vi "HFRR ADV v043.vi"() -> ()   [LabVIEW 2025] (continued)
              n2247 = Fract/Exp String To Number(string=w2642) -> (number=w2638:dbl)  [unwired: 3 in, 1 out]
              n2248 = Fract/Exp String To Number(string=w2632) -> (number=w2635:dbl)  [unwired: 3 in, 1 out]
              n2249 = Add(x=w2635, y=0.0) -> (x+y=w2631:dbl)
            }
            n2250 = Delete From Array(array=w2497, index=0) -> (array with subset deleted=w2470:dbl[])  [unwired: 1 in, 1 out]
            n2251 = Delete From Array(array=w2560, index=0) -> (array with subset deleted=w2533:dbl[])  [unwired: 1 in, 1 out]
            n2252 = Delete From Array(array=w2540, index=0) -> (array with subset deleted=w2528:dbl[])  [unwired: 1 in, 1 out]
            n2253 = Delete From Array(array=w2558, index=0) -> (array with subset deleted=w2559:dbl[])  [unwired: 1 in, 1 out]
            n2254 = call-poly <vilib>:"Mean.vi"("X"=w2470) -> ("mean"=→"КОФ2 4":dbl)  [unwired: 1 out]
            n2255 = call-poly <vilib>:"Mean.vi"("X"=w2533) -> ("mean"=→"КОФ3":dbl)  [unwired: 1 out]
            n2256 = call-poly <vilib>:"Mean.vi"("X"=w2528) -> ("mean"=→"CP3":dbl)  [unwired: 1 out]
            n2257 = Delete From Array(array=w2522, index=0) -> (array with subset deleted=w2449:dbl[])  [unwired: 1 in, 1 out]
            n2258 = Delete From Array(array=w2461, index=0) -> (array with subset deleted=w2448:dbl[])  [unwired: 1 in, 1 out]
            n2259 = Delete From Array(array=w2501, index=0) -> (array with subset deleted=w2472:dbl[])  [unwired: 1 in, 1 out]
            n2260 = Delete From Array(array=w2579, index=0) -> (array with subset deleted=w2534:dbl[])  [unwired: 1 in, 1 out]
            n2261 = Delete From Array(array=w2545, index=0) -> (array with subset deleted=w2530:dbl[])  [unwired: 1 in, 1 out]
            "array w/ subset deleted" <- w2530
            n2262 = Delete From Array(array=w2576, index=0) -> (array with subset deleted=w2577:dbl[])  [unwired: 1 in, 1 out]
            n2263 = call-poly <vilib>:"Mean.vi"("X"=w2472) -> ("mean"=→"КОФ2 2":dbl)  [unwired: 1 out]
            n2264 = call-poly <vilib>:"Mean.vi"("X"=w2534) -> ("mean"=→"КОФ1":dbl)  [unwired: 1 out]
            n2265 = Bundle "Bundle"(w2449, w2448) -> (w2454:cluster{dbl[], dbl[]})  [unwired: 1 in]
            n2266 = Bundle "Bundle"(w2449, w2577) -> (w2441:cluster{dbl[], dbl[]})  [unwired: 1 in]
            n2267 = Delete From Array(array=w2456, index=0) -> (array with subset deleted=w2444:dbl[])  [unwired: 1 in, 1 out]
            n2268 = Delete From Array(array=w2457, index=0) -> (array with subset deleted=w2446:dbl[])  [unwired: 1 in, 1 out]
            n2269 = Delete From Array(array=w2567, index=0) -> (array with subset deleted=w2568:dbl[])  [unwired: 1 in, 1 out]
            n2270 = Delete From Array(array=w2455, index=0) -> (array with subset deleted=w2442:dbl[])  [unwired: 1 in, 1 out]
            n2271 = Delete From Array(array=w2549, index=0) -> (array with subset deleted=w2550:dbl[])  [unwired: 1 in, 1 out]
            n2272 = Delete From Array(array=w2574, index=0) -> (array with subset deleted=w2480:dbl[])  [unwired: 1 in, 1 out]
            n2273 = Delete From Array(array=w2520, index=0) -> (array with subset deleted=w2476:dbl[])  [unwired: 1 in, 1 out]
            n2274 = Delete From Array(array=w2556, index=0) -> (array with subset deleted=w2478:dbl[])  [unwired: 1 in, 1 out]
            n2275 = Delete From Array(array=w2516, index=0) -> (array with subset deleted=w2474:dbl[])  [unwired: 1 in, 1 out]
            n2276 = Delete From Array(array=w2565, index=0) -> (array with subset deleted=w2479:dbl[])  [unwired: 1 in, 1 out]
            n2277 = Delete From Array(array=w2518, index=0) -> (array with subset deleted=w2475:dbl[])  [unwired: 1 in, 1 out]
            n2278 = Delete From Array(array=w2499, index=0) -> (array with subset deleted=w2471:dbl[])  [unwired: 1 in, 1 out]
            n2279 = Delete From Array(array=w2543, index=0) -> (array with subset deleted=w2529:dbl[])  [unwired: 1 in, 1 out]
            n2280 = Delete From Array(array=w2570, index=0) -> (array with subset deleted=w2531:dbl[])  [unwired: 1 in, 1 out]
            n2281 = Delete From Array(array=w2547, index=0) -> (array with subset deleted=w2477:dbl[])  [unwired: 1 in, 1 out]
            n2282 = Delete From Array(array=w2514, index=0) -> (array with subset deleted=w2473:dbl[])  [unwired: 1 in, 1 out]
            n2283 = Delete From Array(array=w2495, index=0) -> (array with subset deleted=w2469:dbl[])  [unwired: 1 in, 1 out]
            n2284 = Delete From Array(array=w2539, index=0) -> (array with subset deleted=w2527:dbl[])  [unwired: 1 in, 1 out]
            n2285 = Delete From Array(array=w2552, index=0) -> (array with subset deleted=w2532:dbl[])  [unwired: 1 in, 1 out]
            n2286 = Delete From Array(array=w2562, index=0) -> (array with subset deleted=w2445:dbl[])  [unwired: 1 in, 1 out]
            n2287 = Delete From Array(array=w2572, index=0) -> (array with subset deleted=w2447:dbl[])  [unwired: 1 in, 1 out]
            n2288 = Delete From Array(array=w2554, index=0) -> (array with subset deleted=w2443:dbl[])  [unwired: 1 in, 1 out]
            n2289 = Bundle "Bundle"(w2449, w2480) -> (w2467:cluster{dbl[], dbl[]})  [unwired: 1 in]
            n2290 = Bundle "Bundle"(w2449, w2534) -> (w2468:cluster{dbl[], dbl[]})  [unwired: 1 in]
            n2291 = Bundle "Bundle"(w2480, w2476) -> (w2482:cluster{dbl[], dbl[]})  [unwired: 1 in]
            n2292 = Bundle "Bundle"(w2445, w2444) -> (w2452:cluster{dbl[], dbl[]})  [unwired: 1 in]
            n2293 = Bundle "Bundle"(w2478, w2474) -> (w2484:cluster{dbl[], dbl[]})  [unwired: 1 in]
            n2294 = Bundle "Bundle"(w2445, w2478) -> (w2588:cluster{dbl[], dbl[]})  [unwired: 1 in]
            n2295 = Bundle "Bundle"(w2445, w2474) -> (w2512:cluster{dbl[], dbl[]})  [unwired: 1 in]
            n2296 = Bundle "Bundle"(w2445, w2533) -> (w2598:cluster{dbl[], dbl[]})  [unwired: 1 in]
            n2297 = Bundle "Bundle"(w2445, w2528) -> (w2536:cluster{dbl[], dbl[]})  [unwired: 1 in]
            n2298 = Bundle "Bundle"(w2445, w2559) -> (w2583:cluster{dbl[], dbl[]})  [unwired: 1 in]
            n2299 = Bundle "Bundle"(w2479, w2475) -> (w2483:cluster{dbl[], dbl[]})  [unwired: 1 in]
            n2300 = Bundle "Bundle"(w2447, w2446) -> (w2453:cluster{dbl[], dbl[]})  [unwired: 1 in]
            n2301 = Bundle "Bundle"(w2447, w2479) -> (w2590:cluster{dbl[], dbl[]})  [unwired: 1 in]
            n2302 = Bundle "Bundle"(w2447, w2475) -> (w2513:cluster{dbl[], dbl[]})  [unwired: 1 in]
            n2303 = Bundle "Bundle"(w2447, w2529) -> (w2537:cluster{dbl[], dbl[]})  [unwired: 1 in]
            n2304 = Bundle "Bundle"(w2447, w2531) -> (w2599:cluster{dbl[], dbl[]})  [unwired: 1 in]
            n2305 = Bundle "Bundle"(w2447, w2568) -> (w2581:cluster{dbl[], dbl[]})  [unwired: 1 in]
            n2306 = Bundle "Bundle"(w2477, w2473) -> (w2485:cluster{dbl[], dbl[]})  [unwired: 1 in]
            n2307 = Bundle "Bundle"(w2443, w2442) -> (w2451:cluster{dbl[], dbl[]})  [unwired: 1 in]
            n2308 = Bundle "Bundle"(w2443, w2477) -> (w2589:cluster{dbl[], dbl[]})  [unwired: 1 in]
            n2309 = Bundle "Bundle"(w2443, w2473) -> (w2511:cluster{dbl[], dbl[]})  [unwired: 1 in]
            n2310 = Bundle "Bundle"(w2443, w2527) -> (w2535:cluster{dbl[], dbl[]})  [unwired: 1 in]
            n2311 = Bundle "Bundle"(w2443, w2532) -> (w2597:cluster{dbl[], dbl[]})  [unwired: 1 in]
            n2312 = Bundle "Bundle"(w2443, w2550) -> (w2582:cluster{dbl[], dbl[]})  [unwired: 1 in]
            n2313 = call-poly <vilib>:"Mean.vi"("X"=w2530) -> ("mean"=→"CP1":dbl)  [unwired: 1 out]
            n2314 = call-poly <vilib>:"Mean.vi"("X"=w2471) -> ("mean"=→"КОФ2 3":dbl)  [unwired: 1 out]
            n2315 = call-poly <vilib>:"Mean.vi"("X"=w2529) -> ("mean"=→"CP2":dbl)  [unwired: 1 out]
            n2316 = call-poly <vilib>:"Mean.vi"("X"=w2531) -> ("mean"=→"КОФ2":dbl)  [unwired: 1 out]
            n2317 = call-poly <vilib>:"Mean.vi"("X"=w2469) -> ("mean"=→"КОФ2 5":dbl)  [unwired: 1 out]
            n2318 = call-poly <vilib>:"Mean.vi"("X"=w2527) -> ("mean"=→"CP4":dbl)  [unwired: 1 out]
            n2319 = call-poly <vilib>:"Mean.vi"("X"=w2532) -> ("mean"=→"КОФ4":dbl)  [unwired: 1 out]
            n2320 = Bundle "Bundle"(w2449, w2476) -> (w2440:cluster{dbl[], dbl[]})  [unwired: 1 in]
            n2321 = Bundle "Bundle"(w2449, w2530) -> (w2463:cluster{dbl[], dbl[]})  [unwired: 1 in]
            n2322 = Build Array "Build Array"(w2440, w2463) -> (w2466:cluster{dbl[], dbl[]}[])
            "XY Graph 17" <- w2466
            n2323 = Build Array "Build Array"(w2454, w2453, w2452, w2451) -> (→"Frequency ( Hz )":cluster{dbl[], dbl[]}[])
            n2324 = Build Array "Build Array"(w2482, w2483, w2484, w2485) -> (→"Air Temp ( °C ) vs Humidity ( % RH )":cluster{dbl[], dbl[]}[])
            n2325 = Build Array "Build Array"(w2467, w2590, w2588, w2589) -> (→"Air Temperature  ( °C )":cluster{dbl[], dbl[]}[])
            n2326 = Build Array "Build Array"(w2440, w2513, w2512, w2511) -> (→"Humidity ( %RH )":cluster{dbl[], dbl[]}[])
            n2327 = Build Array "Build Array"(w2468, w2599, w2598, w2597) -> (→"Coefficient Of Friction":cluster{dbl[], dbl[]}[])
            n2328 = Build Array "Build Array"(w2463, w2537, w2536, w2535) -> (→"Sample Temperature ( °C )":cluster{dbl[], dbl[]}[])
            n2329 = Build Array "Build Array"(w2441, w2581, w2583, w2582) -> (→"XY Graph 13":cluster{dbl[], dbl[]}[])
            n2330 = Bundle "Bundle"(w2449, w2472) -> (w2494:cluster{dbl[], dbl[]})  [unwired: 1 in]
            n2331 = Bundle "Bundle"(w2445, w2470) -> (w2492:cluster{dbl[], dbl[]})  [unwired: 1 in]
            n2332 = Bundle "Bundle"(w2447, w2471) -> (w2493:cluster{dbl[], dbl[]})  [unwired: 1 in]
            n2333 = Bundle "Bundle"(w2443, w2469) -> (w2491:cluster{dbl[], dbl[]})  [unwired: 1 in]
            n2334 = Build Array "Build Array"(w2494, w2493, w2492, w2491) -> (→"Stroke ( mm )":cluster{dbl[], dbl[]}[])
            n2335 = local write "XY Graph 16"(w2466) -> ()
          }
          frame #2 {
          }
          frame #3 {
            n2336 = local write "Numeric 8"(0 ("Numeric 8")) -> ()
            n2337 = local write "Numeric 11"(0 ("Numeric 11")) -> ()
            n2338 = local write "Numeric 12"(0 ("Numeric 12")) -> ()
            n2339 = local write "Numeric 13"(0 ("Numeric 13")) -> ()
            n2340 = property on="OPEN" class="Bool (strict)"("Visible"=TRUE) -> ()  [unwired: 2 in, 2 out]
            n2341 = local read "String Control 2"() -> (w2766:string)
            n2342 = local read "String Control 4"() -> (w2765:string)
            n2343 = local read "String Control 6"() -> (w2764:string)
            n2344 = local read "String Control 8"() -> (w2763:string)
            n2345 = Match Pattern(string=w2766, regular expression="Samples / cycle :- ") -> (after substring=w2780:string)  [unwired: 1 in, 3 out]
            n2346 = Match Pattern(string=w2766, regular expression="Frequency :- ") -> (after substring=w2799:string)  [unwired: 1 in, 3 out]
            n2347 = Match Pattern(string=w2765, regular expression="Samples / cycle :- ") -> (after substring=w2776:string)  [unwired: 1 in, 3 out]
            n2348 = Match Pattern(string=w2765, regular expression="Frequency :- ") -> (after substring=w2794:string)  [unwired: 1 in, 3 out]
            n2349 = Match Pattern(string=w2764, regular expression="Samples / cycle :- ") -> (after substring=w2772:string)  [unwired: 1 in, 3 out]
            n2350 = Match Pattern(string=w2764, regular expression="Frequency :- ") -> (after substring=w2789:string)  [unwired: 1 in, 3 out]
            n2351 = Match Pattern(string=w2763, regular expression="Samples / cycle :- ") -> (after substring=w2768:string)  [unwired: 1 in, 3 out]
            n2352 = Match Pattern(string=w2763, regular expression="Frequency :- ") -> (after substring=w2784:string)  [unwired: 1 in, 3 out]
            n2353 = String Subset(string=w2780, length (rest)=6 ("length (rest)")) -> (substring=w2782:string)  [unwired: 1 in]
            n2354 = String Subset(string=w2799, length (rest)=9 ("length (rest)")) -> (substring=w2801:string)  [unwired: 1 in]
            n2355 = String Subset(string=w2776, length (rest)=6 ("length (rest)")) -> (substring=w2778:string)  [unwired: 1 in]
            n2356 = String Subset(string=w2794, length (rest)=9 ("length (rest)")) -> (substring=w2796:string)  [unwired: 1 in]
            n2357 = String Subset(string=w2772, length (rest)=6 ("length (rest)")) -> (substring=w2774:string)  [unwired: 1 in]
            n2358 = String Subset(string=w2789, length (rest)=9 ("length (rest)")) -> (substring=w2791:string)  [unwired: 1 in]
            n2359 = String Subset(string=w2768, length (rest)=6 ("length (rest)")) -> (substring=w2770:string)  [unwired: 1 in]
            n2360 = String Subset(string=w2784, length (rest)=9 ("length (rest)")) -> (substring=w2786:string)  [unwired: 1 in]
            n2361 = Fract/Exp String To Number(string=w2782) -> (number=w2762:dbl)  [unwired: 3 in, 1 out]
            n2362 = Fract/Exp String To Number(string=w2801) -> (number=w2802:dbl)  [unwired: 3 in, 1 out]
            n2363 = Fract/Exp String To Number(string=w2778) -> (number=w2761:dbl)  [unwired: 3 in, 1 out]
            n2364 = Fract/Exp String To Number(string=w2796) -> (number=w2797:dbl)  [unwired: 3 in, 1 out]
            n2365 = Fract/Exp String To Number(string=w2774) -> (number=w2760:dbl)  [unwired: 3 in, 1 out]
            n2366 = Fract/Exp String To Number(string=w2791) -> (number=w2792:dbl)  [unwired: 3 in, 1 out]
            n2367 = Fract/Exp String To Number(string=w2770) -> (number=w2759:dbl)  [unwired: 3 in, 1 out]
            n2368 = Fract/Exp String To Number(string=w2786) -> (number=w2787:dbl)  [unwired: 3 in, 1 out]
            n2369 = local write "sample1"(w2762) -> ()
            n2370 = local write "freq1"(w2802) -> ()
            n2371 = local write "sample2"(w2761) -> ()
            n2372 = local write "freq2"(w2797) -> ()
            n2373 = local write "sample3"(w2760) -> ()
            n2374 = local write "freq3"(w2792) -> ()
            n2375 = local write "sample4"(w2759) -> ()
            n2376 = local write "freq 4"(w2787) -> ()
          }
        }
      }
    }
    n2377 = case shown="True" w2360 {
      selector: w2360 -> [_ w2379]
      frame False {
      }
      frame True {
        n2378 = Not(x=w2379) -> (.not. x?=w2375:bool)
        n2379 = local write "service 3"(w2375) -> ()
        n2380 = local write "OPEN 6"(w2375) -> ()
        n2381 = call <vilib>:"System Exec.vi"("wait until completion? (T)"=TRUE, "command line"="C:\\LAB-IQ\\Scar View.exe") -> ("error out"=→"error out 5":errorcluster)  [unwired: 6 in, 3 out]
      }
    }
    n2382 = case shown="\"Acquire\", Default" w2369 {
      frame "Acquire", Default {
        # "Elapsed time\ncof\nstroke\nAir temp\nTemp\nHumidity"
        n2383 = disable-structure shown="Disabled" {
          frame Disabled {
            n2384 = local read "Flag"() -> (w3078:dbl)
            n2385 = local read "RUN"() -> (w3075:bool)
            n2386 = Not(x=w3075) -> (.not. x?=w3074:bool)
            n2387 = Equal?(x=w3078, y=10.0) -> (x = y?=w3076:bool)
            n2388 = And(x=w3076, y=w3074) -> (x .and. y?=w3073:bool)
            n2389 = case shown="True" w3073 {
              frame False {
              }
              frame True {
                w3079 = FALSE ("Heater Button")
                n2390 = local write "Humidity"(w3079) -> ()
                n2391 = local write "Heater Button"(w3079) -> ()
              }
            }
          }
          frame Enabled {
          }
        }
        n2392 = disable-structure shown="Disabled" {
          frame Disabled {
            n2393 = case shown="True" {
              selector: _ -> [_ _]
              frame False {
              }
              frame True {
                w3124 = TRUE ("Heater")
                n2394 = local write "Humidity"(w3124) -> ()
                n2395 = local write "Heater Button"(w3124) -> ()
                n2396 = local read "TEST STANDARD"() -> (w3127:T3)
                n2397 = local read "TEST STANDARD"() -> (w3122:T3)
                n2398 = Equal?(x=w3127, y=enum16{"ASTM D6079", "ISO 12156", "Custom"}."ISO 12156" ("Test Standard")) -> (x = y?=w3125:bool)
                n2399 = Equal?(x=w3122, y=enum16{"ASTM D6079", "ISO 12156", "Custom"}."ASTM D6079" ("Test Standard")) -> (x = y?=w3121:bool)
                n2400 = case shown="True" w3125 {
                  frame False {
                  }
                  frame True {
                    n2401 = local write "airtempflg"(FALSE ("airtempflg")) -> ()
                    n2402 = local write item#-1(TRUE ("Heater")) -> ()
                  }
                }
                n2403 = case shown="True" w3121 {
                  frame False {
                  }
                  frame True {
                    n2404 = local write "airtempflg"(TRUE ("airtempflg")) -> ()
                    n2405 = local write item#-1(FALSE ("Heater")) -> ()
                  }
                }
              }
            }
          }
          frame Enabled {
          }
        }
        n2406 = stacked-sequence {
          frame #0 {
            n2407 = case shown="True" "RST FF" {
              frame False {
              }
              frame True {
                w3141 = 0.0 ("X Scale.Range:Maximum")
                n2408 = property on="Frictional Force ( N )" class="WFChart (strict)"("XScale.Maximum"=600.0 ("X Scale.Range:Maximum"), "XScale.Minimum"=w3141, "YScale.Maximum"=10.0 ("Y Scale.Range:Maximum"), "YScale.Minimum"=w3141) -> ()  [unwired: 2 in, 2 out]
              }
            }
          }
          frame #1 {
            n2409 = case shown="True" "RST TEMP" {
              frame False {
              }
              frame True {
                n2410 = property on="Temperature ( Deg C )" class="WFChart (strict)"("XScale.Minimum"=0.0 ("X Scale.Range:Minimum"), "XScale.Maximum"=600.0 ("X Scale.Range:Maximum"), "YScale.Minimum"=0.0 ("Y Scale.Range:Minimum"), "YScale.Maximum"=100.0 ("Y Scale.Range:Maximum")) -> ()  [unwired: 2 in, 2 out]
              }
            }
          }
          frame #2 {
            n2411 = case shown="True" "RSTCOF" {
              frame False {
              }
              frame True {
                n2412 = property on="Coefficient of Friction" class="WFChart (strict)"("XScale.Minimum"=0.0 ("X Scale.Range:Minimum"), "XScale.Maximum"=600.0 ("X Scale.Range:Maximum"), "YScale.Maximum"=1.0 ("X Scale.Range:Minimum"), "YScale.Minimum"=0.0 ("X Scale.Range:Minimum")) -> ()  [unwired: 2 in, 2 out]
              }
            }
          }
          frame #3 {
            n2413 = case shown="True" "RSTCOF 2" {
              frame False {
              }
              frame True {
                (unwired) 100.0 ("Y Scale.Range:Maximum")
                (unwired) 0.0 ("Y Scale.Range:Minimum")
                (unwired) 600.0 ("X Scale.Range:Maximum")
                (unwired) 0.0 ("X Scale.Range:Minimum")
              }
            }
          }
          frame #4 {
            n2414 = case shown="True" "RSTCOF 3" {
              frame False {
              }
              frame True {
                n2415 = property on="Electrical Contact Resistance ( % )" class="WFChart (strict)"("XScale.Minimum"=0.0 ("X Scale.Range:Minimum"), "XScale.Maximum"=600.0 ("X Scale.Range:Maximum"), "YScale.Minimum"=0.0 ("Y Scale.Range:Minimum"), "YScale.Maximum"=100.0 ("Y Scale.Range:Maximum")) -> ()  [unwired: 2 in, 2 out]
              }
            }
          }
        }
        n2416 = local read "RUN"() -> (w3068:bool)
        n2417 = case shown="False" w3068 {
          frame False {
          }
          frame True {
          }
        }
        n2418 = local read "RUN"() -> (w3072:bool)
        n2419 = case shown="False" w3072 {
          tunnel: [FALSE ("TEST RUNNING") TRUE ("TEST RUNNING")] -> w3071
          frame False {
            w3160 = 0.0 ("Flag")
            n2420 = local write "Elapsed time"(0.0 ("elapsedtime")) -> ()
            n2421 = local write "Time Remaining"(w3160) -> ()
            n2422 = local write "Flag"(w3160) -> ()
            n2423 = local write "Remaining Time"(w3160) -> ()
          }
          frame True {
            n2424 = local write "Flag"(10.0 ("Flag")) -> ()
          }
        }
        n2425 = local read "AIR TEMP"() -> (w3066:dbl)
        n2426 = Greater Or Equal?(x=w3066, y=15.0) -> (x >= y?=w3067:bool)
        "powstat" <- w3067
        n2427 = case shown="True" "Save & Continue" {
          frame False {
          }
          frame True {
            n2428 = local read "USER ID"() -> (w3464:string)
            n2429 = local read "FILE"() -> (w3472:string)
            n2430 = String Length(string=w3472) -> (length=w3470:i32)
            n2431 = String Length(string=w3464) -> (length=w3467:i32)
            n2432 = Greater?(x=w3470, y=0) -> (0:w3469:bool)
            n2433 = Greater?(x=w3467, y=0) -> (0:w3466:bool)
            n2434 = And(x=w3469, y=w3466) -> (x .and. y?=w3465:bool)
            n2435 = case shown="True" w3465 {
              frame False {
                n2436 = stacked-sequence {
                  frame #0 {
                    n2437 = One Button Dialog(message="Please Enter a File Name and Operator ID to save data !", button name ("OK")="Ok") -> ()  [unwired: 1 out]
                  }
                  frame #1 {
                    n2438 = local write "Save & Continue"(FALSE ("OK Button")) -> ()
                  }
                }
                n2439 = local write "Save & Continue"(FALSE ("OK Button")) -> ()
              }
              frame True {
                n2440 = stacked-sequence {
                  frame #0 {
                    n2441 = local read "FILE"() -> (w3478:string)
                    n2442 = call "file check.vi"("file name in"=w3478) -> ("file name out"=w3477:string)  [unwired: 9 in, 1 out]
                    n2443 = call <vilib>:"Application Directory.vi"() -> ("Application Directory"=w3488:path)
                    n2444 = Build Path(base path=w3488, name or relative path="data") -> (appended path=w3487:path)
                    n2445 = call <vilib>:"Trim Whitespace.vi"("string"=w3477) -> ("trimmed string"=w3485:string)  [unwired: 1 in]
                    n2446 = call <vilib>:"Trim Whitespace.vi"("string"=w3477) -> ("trimmed string"=w3486:string)  [unwired: 1 in]
                    n2447 = List Folder(path=w3487) -> (folder names=w3483:string[])  [unwired: 3 in, 3 out]
                    n2448 = Match Pattern(string=w3485, regular expression="_(") -> (before substring=w3482:string)  [unwired: 1 in, 3 out]
                    n2449 = for {
                      tunnel: w3483 -> [w3497] mode=indexing
                      tunnel: w3482 -> [w3495]
                      shift-right: [w3493] -> w3480
                      shift-left: bool[] [] -> [w3494]
                      n2450 = Match Pattern(string=w3497, regular expression="_(") -> (before substring=w3496:string)  [unwired: 1 in, 3 out]
                      n2451 = Equal?(x=w3496, y=w3495) -> (x = y?=w3492:bool)
                      n2452 = case shown="True" w3492 {
                        tunnel: w3492 -> [_ w3500]
                        tunnel: w3494 -> [w3499 w3502]
                        tunnel: [w3499 w3501] -> w3493
                        frame False {
                        }
                        frame True {
                          n2453 = Insert Into Array(array=w3502, new element=w3500) -> (w3501:bool[])  [unwired: 1 in]
                        }
                      }
                    }
                    n2454 = Equal?(x=w3483, y=w3482) -> (x = y?=w3491:bool[])
                    n2455 = Or Array Elements(Boolean array=w3491) -> (logical OR=w3490:bool)
                    n2456 = Array Size(array=w3480) -> (size(s)=w3479:i32)
                    n2457 = case shown="True" w3490 {
                      tunnel: w3486 -> [_ w3510]
                      tunnel: w3479 -> [_ w3503]
                      frame False {
                      }
                      frame True {
                        n2458 = Number To Decimal String(number=w3503) -> (decimal integer string=w3506:string)  [unwired: 1 in]
                        n2459 = Search/Split String(string=w3510, search string/char (-)="_(" ("regular expression")) -> (substring before match=w3508:string)  [unwired: 1 in, 2 out]
                        n2460 = Concatenate Strings(w3508, "_(" ("regular expression"), w3506, ")" ("regular expression")) -> (w3504:string)
                        n2461 = local write "FILE"(w3504) -> ()
                      }
                    }
                  }
                  frame #1 {
                    w3513 = 0.0
                    w3526 = cluster{"y":dbl, dbl, "y":dbl}[] [] ("History Data")
                    w3527 = FALSE ("Heater Button")
                    (unwired) ")!" ("string")
                    (unwired) ")" ("string")
                    w3525 = dbl[] [] ("History Data")
                    w3531 = "\r"
                    # "C:\\WinDucom\\Data\\"
                    # "C:\\LAB-IQ-NXT\\data"
                    n2462 = local write "Humidity ( %RH )"(w3513) -> ()
                    n2463 = local write "Frequency ( Hz )"(w3513) -> ()
                    n2464 = local write "Stroke 3"(w3513) -> ()
                    n2465 = local write "speedop"(0.0 ("PIDclk 2")) -> ()
                    n2466 = local write "Set Temp 2"(65.0 ("Set Temp 2")) -> ()
                    n2467 = local write "AIR TEMP"(w3513) -> ()
                    n2468 = local write "clk"(0.0 ("clk")) -> ()
                    n2469 = local write "Stroke 4"(w3513) -> ()
                    n2470 = local write "COF 2"(w3513) -> ()
                    n2471 = local write "TEMP"(w3513) -> ()
                    n2472 = local write "ecr 3"(w3513) -> ()
                    n2473 = local write "FF 3"(w3513) -> ()
                    n2474 = local write "FF 2"(w3513) -> ()
                    n2475 = property on="Coefficient of Friction" class="WFChart (strict)"("History Data"=w3525) -> ()  [unwired: 2 in, 2 out]
                    n2476 = property on="Coefficient of Friction" class="WFChart (strict)"("History Data"=w3525) -> ()  [unwired: 2 in, 2 out]
                    n2477 = property on="Frictional Force ( N )" class="WFChart (strict)"("History Data"=w3525) -> ()  [unwired: 2 in, 2 out]
                    n2478 = property on="Electrical Contact Resistance ( % )" class="WFChart (strict)"("History Data"=w3525) -> ()  [unwired: 2 in, 2 out]
                    n2479 = property on="Electrical Contact Resistance ( % )" class="WFChart (strict)"("History Data"=w3525) -> ()  [unwired: 2 in, 2 out]
                    n2480 = property on="Temperature ( Deg C )" class="WFChart (strict)"("History Data"=w3525) -> ()  [unwired: 2 in, 2 out]
                    n2481 = property on="Frictional Force ( N )" class="WFChart (strict)"("History Data"=w3525) -> ()  [unwired: 2 in, 2 out]
                    n2482 = property on="Coefficient of Friction" class="WFChart (strict)"("History Data"=w3525) -> ()  [unwired: 2 in, 2 out]
                    n2483 = property on="Frictional Force ( N )" class="WFChart (strict)"("History Data"=w3525) -> ()  [unwired: 2 in, 2 out]
                    n2484 = property on="Electrical Contact Resistance ( % )" class="WFChart (strict)"("History Data"=w3525) -> ()  [unwired: 2 in, 2 out]
                    n2485 = property on="Temperature ( Deg C )" class="WFChart (strict)"("History Data"=w3525) -> ()  [unwired: 2 in, 2 out]
                    n2486 = property on="Stroke ( mm )" class="WFChart (strict)"("History Data"=w3526) -> ()  [unwired: 2 in, 2 out]
                    n2487 = property on="Stroke ( mm )" class="WFChart (strict)"("History Data"=w3526) -> ()  [unwired: 2 in, 2 out]
                    n2488 = local write "Humidity"(w3527) -> ()
                    n2489 = local write "Heater Button"(w3527) -> ()
                    n2490 = local read "FILE"() -> (w3521:string)
                    n2491 = disable-structure shown="Enabled" {
                      disable-tunnel: [w3565 _] -> w3512
                      frame Enabled {
                        n2492 = local read "NORMAL LOAD"() -> (w3565:dbl)
                      }
                      frame Disabled {
                      }
                    }
                    n2493 = call "file check.vi"("file name in"=w3521) -> ("error out"=w3524:errorcluster, "file name out"=w3518:string)  [unwired: 9 in]
                    n2494 = call "FILE PATH CREATION.vi"("error in"=w3524, "FILE NAME :"=w3518) -> ("FILE OUT"=w3517:path)  [unwired: 8 in, 1 out]
                    n2495 = Concatenate Strings(w3518, ".dgf" ("Substring")) -> (w3523:string)
                    n2496 = Concatenate Strings(w3518, ".duf" ("Substring")) -> (w3519:string)
                    n2497 = Multiply(x=w3512, y=1.0) -> (x*y=w3544:dbl)
                    n2498 = Build Path(base path=w3517, name or relative path=w3523) -> (appended path=w3516:path)
                    n2499 = Build Path(base path=w3517, name or relative path=w3519) -> (appended path=w3515:path)
                    n2500 = Number To Fractional String(number=w3544, width (-)=i16 5, precision (6)=i16 2) -> (F-format string=w3552:string)  [unwired: 1 in]
                    n2501 = local read "tested by"() -> (w3511:string)
                    n2502 = local read "Fuel Discription :"() -> (w3540:string)
                    n2503 = local read "Batch Ref Num :"() -> (w3529:string)
                    n2504 = Get Date/Time String(date format (0)=enum16{"short", "long", "abbreviated"}."short") -> (date string=w3563:string, time string=w3560:string)  [unwired: 2 in]
                    n2505 = local read "Remarks :"() -> (w3539:string)
                    n2506 = Concatenate Strings("Load :- " ("Substring"), w3552, " grams ," ("Substring")) -> (w3551:string)
                    n2507 = local read "String 41"() -> (w3532:string)
                    n2508 = Concatenate Strings(w3540) -> (w3541:string)
                    n2509 = Concatenate Strings(w3529) -> (w3528:string)
                    n2510 = Concatenate Strings(w3511) -> (w3535:string)
                    n2511 = Concatenate Strings("(" ("Substring"), w3563, ")" ("Substring"), w3560) -> (w3534:string)
                    "concatenated string" <- w3534
                    n2512 = Concatenate Strings(w3539, "," ("string")) -> (w3538:string)
                    n2513 = Concatenate Strings("  TIME;      COF;       STROKE;     AIR TEMP;  TEMP;  HUMIDITY;  ECR; PID-OUT; FREQUENCY" ("Substring"), "\r") -> (w3547:string)
                    n2514 = Concatenate Strings(w3532, w3531, "Fuel Discription :-" ("Substring"), w3541, w3531, w3551, w3531, "Batch Ref Num :-" ("Substring"), w3528, w3531, " Remarks :- " ("Substring"), w3538, w3531, " Date :- " ("Substring"), w3534, w3531, "Tested By :-" ("Substring"), w3535) -> (w3545:string)
                    "REMARKS" <- w3545
                    n2515 = call <vilib>:"Write Characters To File.vi"("append to file? (new file:F)"=FALSE, "character string"=w3547, "file path (dialog if empty)"=w3516) -> ()  [unwired: 2 in, 1 out]
                    n2516 = call <vilib>:"Write Characters To File.vi"("append to file? (new file:F)"=FALSE, "character string"=w3545, "file path (dialog if empty)"=w3515) -> ()  [unwired: 2 in, 1 out]
                  }
                  frame #2 {
                    n2517 = local write "Cycles elapsed"(0 ("Cycles elapsed")) -> ()
                    n2518 = local write "cyclecount"(0 ("cyclecount")) -> ()
                    n2519 = local write "Save & Continue"(FALSE ("OK")) -> ()
                    n2520 = local write "autostrtflg"(TRUE ("autostrtflg")) -> ()
                    n2521 = local write "Save"(FALSE ("Save")) -> ()
                    n2522 = Get Date/Time In Seconds() -> (seconds since 1Jan1904=w3570:timestamp)
                    n2523 = To Double Precision Float(number=w3570) -> (double precision float=w3569:dbl)
                    n2524 = local write "acq timer"(w3569) -> ()
                    n2525 = One Button Dialog(message="Please ensure sample is mounted properly and machine is ready in all aspects for testing !", button name ("OK")="Ok") -> ()  [unwired: 1 out]
                  }
                  frame #3 {
                    n2526 = stacked-sequence {
                      frame #0 {
                        n2527 = local write "Main Dashboard Buttons"(T1."Dashboard" ("Main Dashboard Buttons")) -> ()
                        n2528 = local write "Main Tab"(T2."Acquire" ("Main Tab")) -> ()
                      }
                      frame #1 {
                        n2529 = local write "EVENT LOG"("" ("EVENT LOG")) -> ()
                      }
                      frame #2 {
                        n2530 = Wait (ms)(milliseconds to wait=u32 50) -> ()  [unwired: 1 out]
                      }
                      frame #3 {
                        n2531 = disable-structure shown="Disabled" {
                          frame Disabled {
                            n2532 = local read "EVENT LOG"() -> (w3582:string)
                            n2533 = call "Event Log.vi"("Content"="Test Details", "EVENT LOG"=w3582) -> ("EVENT LOG"=w3581:string)  [unwired: 8 in, 1 out]
                            n2534 = local write "EVENT LOG"(w3581) -> ()
                          }
                          frame Enabled {
                          }
                        }
                      }
                      frame #4 {
                        n2535 = Wait (ms)(milliseconds to wait=u32 50) -> ()  [unwired: 1 out]
                      }
                      frame #5 {
                        n2536 = local read "FILE"() -> (w3584:string)
                        n2537 = Concatenate Strings("File Name :" ("Content"), w3584) -> (w3585:string)
                        n2538 = local read "EVENT LOG"() -> (w3588:string)
                        n2539 = call "Event Log.vi"("Content"=w3585, "EVENT LOG"=w3588) -> ("EVENT LOG"=w3587:string)  [unwired: 8 in, 1 out]
                        n2540 = local write "EVENT LOG"(w3587) -> ()
                      }
                      frame #6 {
                        n2541 = Wait (ms)(milliseconds to wait=u32 50) -> ()  [unwired: 1 out]
                      }
                      frame #7 {
                        n2542 = local read "Batch Ref Num :"() -> (w3590:string)
                        n2543 = Concatenate Strings("Batch Ref No :" ("Content"), w3590) -> (w3591:string)
                        n2544 = local read "EVENT LOG"() -> (w3594:string)
                        n2545 = call "Event Log.vi"("Content"=w3591, "EVENT LOG"=w3594) -> ("EVENT LOG"=w3593:string)  [unwired: 8 in, 1 out]
                        n2546 = local write "EVENT LOG"(w3593) -> ()
                      }
                      frame #8 {
                        n2547 = Wait (ms)(milliseconds to wait=u32 50) -> ()  [unwired: 1 out]
                      }
                      frame #9 {
                        n2548 = local read "tested by"() -> (w3596:string)
                        n2549 = Concatenate Strings("Tested By :" ("Content"), w3596) -> (w3597:string)
                        n2550 = local read "EVENT LOG"() -> (w3600:string)
                        n2551 = call "Event Log.vi"("Content"=w3597, "EVENT LOG"=w3600) -> ("EVENT LOG"=w3599:string)  [unwired: 8 in, 1 out]
                        n2552 = local write "EVENT LOG"(w3599) -> ()
                      }
                      frame #10 {
                        n2553 = Wait (ms)(milliseconds to wait=u32 50) -> ()  [unwired: 1 out]
                      }
                      frame #11 {
                        n2554 = local read "TEST STANDARD"() -> (w3603:T3)
                        n2555 = case shown="\"ASTM D6079\", Default" w3603 {
                          tunnel: ["ASTM D6079" "ISO 12156" "CEC F-096-A-06" "Custom"] -> w3602
                          frame "ASTM D6079", Default {
                          }
                          frame "ISO 12156" {
                          }
                          frame "CEC F-096-A-06" {
                          }
                          frame "Custom" {
                          }
                        }
                        n2556 = Concatenate Strings("Test Standard :" ("Content"), w3602) -> (w3604:string)
                        n2557 = local read "EVENT LOG"() -> (w3607:string)
                        n2558 = call "Event Log.vi"("Content"=w3604, "EVENT LOG"=w3607) -> ("EVENT LOG"=w3606:string)  [unwired: 8 in, 1 out]
                        n2559 = local write "EVENT LOG"(w3606) -> ()
                      }
                      frame #12 {
                        n2560 = Wait (ms)(milliseconds to wait=u32 50) -> ()  [unwired: 1 out]
                      }
                      frame #13 {
                        n2561 = local read "Fuel Discription :"() -> (w3613:string)
                        n2562 = Concatenate Strings("Fuel Description :" ("Content"), w3613) -> (w3614:string)
                        n2563 = local read "EVENT LOG"() -> (w3617:string)
                        n2564 = call "Event Log.vi"("Content"=w3614, "EVENT LOG"=w3617) -> ("EVENT LOG"=w3616:string)  [unwired: 8 in, 1 out]
                        n2565 = local write "EVENT LOG"(w3616) -> ()
                      }
                      frame #14 {
                        n2566 = Wait (ms)(milliseconds to wait=u32 50) -> ()  [unwired: 1 out]
                      }
                      frame #15 {
                        n2567 = local read "Remarks :"() -> (w3619:string)
                        n2568 = Concatenate Strings("Remarks :" ("Content"), w3619) -> (w3620:string)
                        n2569 = local read "EVENT LOG"() -> (w3623:string)
                        n2570 = call "Event Log.vi"("Content"=w3620, "EVENT LOG"=w3623) -> ("EVENT LOG"=w3622:string)  [unwired: 8 in, 1 out]
                        n2571 = local write "EVENT LOG"(w3622) -> ()
                      }
                      frame #16 {
                        n2572 = Wait (ms)(milliseconds to wait=u32 50) -> ()  [unwired: 1 out]
                      }
                      frame #17 {
                        n2573 = local read "USER ID"() -> (w3625:string)
                        n2574 = Concatenate Strings("Operator ID :" ("Content"), w3625) -> (w3627:string)
                        n2575 = local read "EVENT LOG"() -> (w3629:string)
                        n2576 = call "Event Log.vi"("Content"=w3627, "EVENT LOG"=w3629) -> ("EVENT LOG"=w3628:string)  [unwired: 8 in, 1 out]
                        n2577 = local write "EVENT LOG"(w3628) -> ()
                      }
                      frame #18 {
                        n2578 = Wait (ms)(milliseconds to wait=u32 50) -> ()  [unwired: 1 out]
                      }
                      frame #19 {
                        n2579 = disable-structure shown="Disabled" {
                          frame Disabled {
                            n2580 = local read "EVENT LOG"() -> (w3633:string)
                            n2581 = call "Event Log.vi"("Content"="Test Parameter", "EVENT LOG"=w3633) -> ("EVENT LOG"=w3632:string)  [unwired: 8 in, 1 out]
                            n2582 = local write "EVENT LOG"(w3632) -> ()
                          }
                          frame Enabled {
                          }
                        }
                      }
                      frame #20 {
                        n2583 = Wait (ms)(milliseconds to wait=u32 50) -> ()  [unwired: 1 out]
                      }
                      frame #21 {
                        n2584 = local read "Set Hz"() -> (w3637:dbl)
                        n2585 = Number To Fractional String(number=w3637, precision (6)=i16 2) -> (F-format string=w3636:string)  [unwired: 2 in]
                        n2586 = Concatenate Strings("Set Frequency [Hz] :" ("Content"), w3636) -> (w3639:string)
                        n2587 = local read "EVENT LOG"() -> (w3641:string)
                        n2588 = call "Event Log.vi"("Content"=w3639, "EVENT LOG"=w3641) -> ("EVENT LOG"=w3640:string)  [unwired: 8 in, 1 out]
                        n2589 = local write "EVENT LOG"(w3640) -> ()
                      }
                      frame #22 {
                        n2590 = Wait (ms)(milliseconds to wait=u32 50) -> ()  [unwired: 1 out]
                      }
                      frame #23 {
                        n2591 = local read "NORMAL LOAD"() -> (w3644:dbl)
                        n2592 = Number To Fractional String(number=w3644, precision (6)=i16 2) -> (F-format string=w3645:string)  [unwired: 2 in]
                        n2593 = Concatenate Strings("Applied Load [grams] :" ("Content"), w3645) -> (w3647:string)
                        n2594 = local read "EVENT LOG"() -> (w3649:string)
                        n2595 = call "Event Log.vi"("Content"=w3647, "EVENT LOG"=w3649) -> ("EVENT LOG"=w3648:string)  [unwired: 8 in, 1 out]
                        n2596 = local write "EVENT LOG"(w3648) -> ()
                      }
                      frame #24 {
                        n2597 = Wait (ms)(milliseconds to wait=u32 50) -> ()  [unwired: 1 out]
                      }
                      frame #25 {
                        n2598 = local read "Set Strk"() -> (w3652:dbl)
                        n2599 = Number To Fractional String(number=w3652, precision (6)=i16 2) -> (F-format string=w3653:string)  [unwired: 2 in]
                        n2600 = Concatenate Strings("Set Stroke [mm] :" ("Content"), w3653) -> (w3655:string)
                        n2601 = local read "EVENT LOG"() -> (w3657:string)
                        n2602 = call "Event Log.vi"("Content"=w3655, "EVENT LOG"=w3657) -> ("EVENT LOG"=w3656:string)  [unwired: 8 in, 1 out]
                        n2603 = local write "EVENT LOG"(w3656) -> ()
                      }
                      frame #26 {
                        n2604 = Wait (ms)(milliseconds to wait=u32 50) -> ()  [unwired: 1 out]
                      }
                      frame #27 {
                        n2605 = local read "Set Temp"() -> (w3660:dbl)
                        n2606 = Number To Fractional String(number=w3660, precision (6)=i16 2) -> (F-format string=w3661:string)  [unwired: 2 in]
                        n2607 = Concatenate Strings("Set Temperature [deg C] :" ("Content"), w3661) -> (w3663:string)
                        n2608 = local read "EVENT LOG"() -> (w3665:string)
                        n2609 = call "Event Log.vi"("Content"=w3663, "EVENT LOG"=w3665) -> ("EVENT LOG"=w3664:string)  [unwired: 8 in, 1 out]
                        n2610 = local write "EVENT LOG"(w3664) -> ()
                      }
                      frame #28 {
                        n2611 = Wait (ms)(milliseconds to wait=u32 50) -> ()  [unwired: 1 out]
                      }
                      frame #29 {
                        n2612 = local read "Set Rh"() -> (w3668:dbl)
                        n2613 = Number To Fractional String(number=w3668, precision (6)=i16 2) -> (F-format string=w3669:string)  [unwired: 2 in]
                        n2614 = Concatenate Strings("Set Humidity [%RH] :" ("Content"), w3669) -> (w3671:string)
                        n2615 = local read "EVENT LOG"() -> (w3673:string)
                        n2616 = call "Event Log.vi"("Content"=w3671, "EVENT LOG"=w3673) -> ("EVENT LOG"=w3672:string)  [unwired: 8 in, 1 out]
                        n2617 = local write "EVENT LOG"(w3672) -> ()
                      }
                      frame #30 {
                        n2618 = Wait (ms)(milliseconds to wait=u32 50) -> ()  [unwired: 1 out]
                      }
                      frame #31 {
                        n2619 = local read "test time"() -> (w3676:dbl)
                        n2620 = Number To Fractional String(number=w3676, precision (6)=i16 1) -> (F-format string=w3677:string)  [unwired: 2 in]
                        n2621 = Concatenate Strings("Test Duration [mins] :" ("Content"), w3677) -> (w3679:string)
                        n2622 = local read "EVENT LOG"() -> (w3681:string)
                        n2623 = call "Event Log.vi"("Content"=w3679, "EVENT LOG"=w3681) -> ("EVENT LOG"=w3680:string)  [unwired: 8 in, 1 out]
                        n2624 = local write "EVENT LOG"(w3680) -> ()
                      }
                      frame #32 {
                        w3682 = dbl[] [] ("History Data")
                        w3683 = cluster{"y":dbl, dbl, "y":dbl}[] [] ("History Data")
                        w3684 = FALSE ("Visible")
                        n2625 = property on="Stroke ( mm )" class="WFChart (strict)"("History Data"=w3683) -> ()  [unwired: 2 in, 2 out]
                        n2626 = property on="Temperature ( Deg C )" class="WFChart (strict)"("History Data"=w3682) -> ()  [unwired: 2 in, 2 out]
                        n2627 = property on="Electrical Contact Resistance ( % )" class="WFChart (strict)"("History Data"=w3682) -> ()  [unwired: 2 in, 2 out]
                        n2628 = property on="Coefficient of Friction" class="WFChart (strict)"("History Data"=w3682) -> ()  [unwired: 2 in, 2 out]
                        n2629 = property on="Frictional Force ( N )" class="WFChart (strict)"("History Data"=w3682) -> ()  [unwired: 2 in, 2 out]
                        n2630 = property on="Coefficient of Friction" class="WFChart (strict)"("History Data"=w3682) -> ()  [unwired: 2 in, 2 out]
                        n2631 = property on="Frictional Force ( N )" class="WFChart (strict)"("History Data"=w3682) -> ()  [unwired: 2 in, 2 out]
                        n2632 = property on="Electrical Contact Resistance ( % )" class="WFChart (strict)"("History Data"=w3682) -> ()  [unwired: 2 in, 2 out]
                        n2633 = property on="Stroke ( mm )" class="WFChart (strict)"("History Data"=w3683) -> ()  [unwired: 2 in, 2 out]
                        n2634 = property on="Temperature ( Deg C )" class="WFChart (strict)"("History Data"=w3682) -> ()  [unwired: 2 in, 2 out]
                        n2635 = property on="Service Password Log" class="Str"("Visible"=w3684) -> ()  [unwired: 2 in, 2 out]
                        n2636 = property on="Password 3" class="Clust (strict)"("Visible"=w3684) -> ()  [unwired: 2 in, 2 out]
                      }
                    }
                    "TEST FILE NAM,E SAVED" <- TRUE ("TEST FILE NAM,E SAVED")
                  }
                }
              }
            }
          }
        }
        n2637 = local write "Test \nStatus"(w3071) -> ()
        n2638 = local write "Save"(w3071) -> ()
        n2639 = local read "Main Tab"() -> (w3065:T2)
        n2640 = case shown="True" w3068 {
          frame False {
            n2641 = local read "Rt 3"() -> (w3132:bool)
            n2642 = case shown="True" w3132 {
              frame False {
              }
              frame True {
                n2643 = local write "Rt 3"(FALSE ("Rt 3")) -> ()
              }
            }
            "Rt" <- TRUE ("Rt")
            "Rt 2" <- FALSE ("Rt")
          }
          frame True {
            n2644 = local read "Rt"() -> (w3138:bool)
            n2645 = local write "Rt 2"(TRUE ("Rt 2")) -> ()
            n2646 = case shown="True" w3138 {
              frame False {
              }
              frame True {
                n2647 = local write "Rt"(FALSE ("Rt")) -> ()
              }
            }
            "Rt 3" <- TRUE ("Rt 3")
          }
        }
        n2648 = case shown="\"Acquire\"" w3065 {
          tunnel: w3067 -> [_ w3167]
          frame Default {
            w3166 = 0.0 ("output")
            n2649 = local write "PID-out"(w3166) -> ()
            n2650 = local write "Frequency ( Hz )"(w3166) -> ()
            n2651 = local write "STROKE Initialize"(TRUE ("STROKE Initialize")) -> ()
          }
          frame "Acquire" {
            n2652 = stacked-sequence {
              frame #0 {
                n2653 = local read "Auto Start Test"() -> (w3169:bool)
                n2654 = case shown="True" w3169 {
                  tunnel: "RUN" -> [w3190 w3193]
                  tunnel: [w3190 w3192] -> w3170
                  frame False {
                  }
                  frame True {
                    n2655 = local read "Auto Start Temp"() -> (w3191:bool)
                    n2656 = Or(x=w3193, y=w3191) -> (x .or. y?=w3192:bool)
                  }
                }
                n2657 = local read "clk"() -> (w3189:dbl)
                n2658 = local read "Save"() -> (w3185:bool)
                n2659 = Equal?(x=w3189, y=0.0) -> (x = y?=w3186:bool)
                n2660 = And(x=w3186, y=w3185) -> (x .and. y?=w3187:bool)
                n2661 = Not(x="Engage") -> (.not. x?=w3176:bool)
                n2662 = case shown="False" w3170 {
                  tunnel: [0.0 w3217] -> w3172
                  frame False {
                    (unwired) TRUE ("Visible")
                    n2663 = local read "Auto Start Test"() -> (w3197:bool)
                    n2664 = local write "Start Time"(TRUE ("Start Time")) -> ()
                    n2665 = property on="Stroke 2" class="DigNum (strict)"("Visible"=FALSE) -> ()  [unwired: 2 in, 2 out]
                    n2666 = case shown="False" w3197 {
                      frame False {
                        n2667 = property on="Heater Button" class="Bool (strict)"("DisabledEnum"=T19."Enabled" ("Disabled")) -> ()  [unwired: 2 in, 2 out]
                        n2668 = property on="Humidity" class="Bool (strict)"("DisabledEnum"=T19."Enabled" ("Disabled")) -> ()  [unwired: 2 in, 2 out]
                      }
                      frame True {
                      }
                    }
                    n2669 = case shown="False" "TestCompFlg" {
                      frame False {
                        n2670 = local read "StartFlg"() -> (w3205:bool)
                        n2671 = case shown="True" w3205 {
                          frame False {
                          }
                          frame True {
                            n2672 = stacked-sequence {
                              frame #0 {
                                n2673 = local read "EVENT LOG"() -> (w3209:string)
                                n2674 = call "Event Log.vi"("Content"="Test was interrupted", "EVENT LOG"=w3209) -> ("EVENT LOG"=w3210:string)  [unwired: 8 in, 1 out]
                                n2675 = local write "EVENT LOG"(w3210) -> ()
                                n2676 = property on="RUN" class="Bool (strict)"("Visible"=TRUE) -> ()  [unwired: 2 in, 2 out]
                                n2677 = property on="Auto Start Test" class="Bool (strict)"("Visible"=TRUE) -> ()  [unwired: 2 in, 2 out]
                              }
                              frame #1 {
                                w3213 = FALSE ("StartFlg")
                                n2678 = property on="Heater Button" class="Bool (strict)"("Val(Sgnl)"=FALSE ("Value (Signaling)")) -> ()  [unwired: 2 in, 2 out]
                                n2679 = local write "Heater Button"(w3213) -> ()
                                n2680 = local write "StartFlg"(w3213) -> ()
                                n2681 = local write "Humidity"(w3213) -> ()
                                n2682 = local write "Humidity 2"(TRUE ("Humidity")) -> ()
                              }
                              frame #2 {
                                n2683 = local write "Due Write"("VC;0" ("Command")) -> ()
                              }
                              frame #3 {
                                n2684 = Wait (ms)(milliseconds to wait=u32 1500) -> ()  [unwired: 1 out]
                              }
                              frame #4 {
                                n2685 = local write "Due Write"("HE;0" ("Command")) -> ()
                              }
                            }
                          }
                        }
                      }
                      frame True {
                      }
                    }
                    n2686 = local write "String 14"("Test will autostart once parameters reach the set value." ("String 14")) -> ()
                  }
                  frame True {
                    (unwired) FALSE ("Visible")
                    n2687 = property on="Stroke 2" class="DigNum (strict)"("Visible"=TRUE) -> ()  [unwired: 2 in, 2 out]
                    n2688 = property on="STOP 2" class="Bool (strict)"("Disabled"=u8 2) -> ()  [unwired: 2 in, 2 out]
                    n2689 = local write "String 14"(" Running....." ("String 14")) -> ()
                    n2690 = property on="Heater Button" class="Bool (strict)"("DisabledEnum"=T19."Disabled and Grayed Out" ("Disabled")) -> ()  [unwired: 2 in, 2 out]
                    n2691 = property on="Humidity" class="Bool (strict)"("DisabledEnum"=T19."Disabled and Grayed Out" ("Disabled")) -> ()  [unwired: 2 in, 2 out]
                    n2692 = case shown="True" "Start Time" {
                      selector: "Start Time" -> [_ w3236]
                      frame False {
                      }
                      frame True {
                        n2693 = Not(x=w3236) -> (.not. x?=w3235:bool)
                        n2694 = local write "Start Time"(w3235) -> ()
                        n2695 = local read "EVENT LOG"() -> (w3237:string)
                        n2696 = call "Event Log.vi"("Content"="Test in progress", "EVENT LOG"=w3237) -> ("EVENT LOG"=w3239:string)  [unwired: 8 in, 1 out]
                        n2697 = local write "EVENT LOG"(w3239) -> ()
                      }
                    }
                    n2698 = disable-structure shown="Enabled" {
                      disable-tunnel: [w3228 w3234] -> w3217
                      frame Disabled {
                        n2699 = local read "Set Hz"() -> (w3231:dbl)
                        n2700 = call <vilib>:"Uniform White Noise Waveform.vi"() -> ("signal out"=w3230:waveform(dbl))  [unwired: 10 in, 1 out]
                        n2701 = Random Number (0-1)() -> (number: 0 to 1=w3227:dbl)
                        n2702 = Add(x=w3231, y=w3230) -> (x+y=w3229:waveform(dbl))
                        n2703 = Multiply(x=ext 0.01 ("y"), y=w3227) -> (x*y=w3225:ext)
                        n2704 = Multiply(x=w3229, y=w3225) -> (x*y=w3228:waveform(ext))
                      }
                      frame Enabled {
                        n2705 = call-poly <vilib>:"Random Number (Range).vi"("lower bound (0)"=49.89, "upper bound (100)"=50.8) -> ("number"=w3234:dbl)  [unwired: 9 in]
                      }
                    }
                    "StartFlg" <- TRUE ("StartFlg")
                  }
                }
                n2706 = case shown="True" w3187 {
                  frame False {
                  }
                  frame True {
                    n2707 = local write "clk"(10.0 ("clk")) -> ()
                    n2708 = Get Date/Time In Seconds() -> (seconds since 1Jan1904=w3242:timestamp)
                    n2709 = To Double Precision Float(number=w3242) -> (double precision float=w3240:dbl)
                    n2710 = local write "acq timer"(w3240) -> ()
                    n2711 = local write "act save time"(w3240) -> ()
                  }
                }
                n2712 = call "Elapsed Time"("Time Target (s)"="Countdown", "Reset"=w3176) -> ("Elapsed Time (s)"=w3181:dbl, "Time has Elapsed"=w3179:bool)  [unwired: 10 in, 6 out]
                "Countdown 2" <- w3181
                n2713 = Subtract(x=w3181, y=2.0) -> (x-y=w3184:dbl)
                n2714 = Less?(x=w3184, y="Countdown") -> (x < y?=w3182:bool)
                n2715 = And(x=w3182, y=w3179) -> (x .and. y?=w3178:bool)
                n2716 = case shown="True" w3178 {
                  frame False {
                  }
                  frame True {
                    (unwired) dbl[] [] ("History Data")
                    n2717 = local write "Engage"(FALSE ("Engage")) -> ()
                    n2718 = local write "RUN"(TRUE ("RUN")) -> ()
                    n2719 = local read "Humidity ( %RH )"() -> (→"Rh Before":dbl)
                  }
                }
                n2720 = local read "Test \nStatus"() -> (w3174:bool)
                n2721 = Select(t=w3172, s=w3174, f=0.0) -> (s? t:f=w3173:dbl)
                n2722 = local write "Frequency ( Hz )"(w3173) -> ()
              }
              frame #1 {
                w3265 = 1000000.0 ("x")
                # "HC;1/0\nST;VALUE"
                # "Elapsed time\ncof\nstroke\nAir temp\nTemp\nHumidity"
                # "acq timer\n\nact save time"
                # "convert to microseconds"
                n2723 = local read "COUNT"() -> (w3248:i32)
                n2724 = local read "Rate"() -> (w3261:dbl)
                n2725 = Divide(x=w3265, y=w3261) -> (x/y=w3266:dbl)
                n2726 = Greater Or Equal?(x=w3248, y=250) -> (x >= y?=w3247:bool)
                n2727 = Get Date/Time In Seconds() -> (seconds since 1Jan1904=w3268:timestamp)
                n2728 = case shown="True" w3247 {
                  frame False {
                    n2729 = local read "COUNT"() -> (w3269:i32)
                    n2730 = Increment(x=w3269) -> (x+1=w3270:i32)
                    n2731 = local write "COUNT"(w3270) -> ()
                  }
                  frame True {
                    n2732 = local write "COUNT"(0 ("COUNT")) -> ()
                  }
                }
                n2733 = local read "Samplingtime 2"() -> (w3246:dbl)
                n2734 = local read "act save time"() -> (w3263:dbl)
                n2735 = Divide(x=w3266, y=w3265) -> (x/y=w3264:dbl)
                n2736 = To Double Precision Float(number=w3268) -> (double precision float=w3257:dbl)
                n2737 = Add(x=w3263, y=w3246) -> (x+y=w3262:dbl)
                n2738 = local read "acq timer"() -> (w3267:dbl)
                n2739 = local read "COUNT"() -> (w3250:i32)
                n2740 = Greater Or Equal?(x=w3257, y=w3262) -> (x >= y?=w3245:bool)